vi "Dresden R2R Sputter 03.02.2018 IY24.vi"() -> ()   [LabVIEW 2009] (continued)
                                n25886 = Or(x=w31134, y=w31133) -> (x .or. y?=w31132:bool)
                                }
                                }
                                frame #1 {
                                }
                                }
                                }
                                frame #8 {
                                n25887 = local read "Semi"() -> (w31142:bool)
                                n25888 = case shown="False" w31142 {
                                frame #0 {
                                n25889 = while {
                                i -> [w31143]
                                stop <- w31147 stop-if-true
                                n25890 = Greater?(x=w31143, y=50) -> (0:w31145:bool)
                                n25891 = case shown="True" w31145 {
                                frame #0 {
                                }
                                frame #1 {
                                n25892 = local write "Error Message"("Transfer process was\ncancelled.Please check left limit sensor." ("Error Message")) -> ()
                                n25893 = local write "Semi"(TRUE ("Semi")) -> ()
                                }
                                }
                                n25894 = local read "Cnt_Left_limit_di"() -> (w31149:bool)
                                n25895 = case shown="False" w31149 {
                                tunnel: [FALSE ("Ch1_pet_cool_up_do") TRUE ("Ch1_pet_cool_up_do")] -> w31148
                                frame #0 {
                                n25896 = local write "Cnt_Left_limit_do"(TRUE ("Ch1_pet_cool_up_do")) -> ()
                                n25897 = Wait Until Next ms Multiple(millisecond multiple=u32 200) -> ()  [unwired: 1 out]
                                }
                                frame #1 {
                                }
                                }
                                n25898 = local read "Semi"() -> (w31146:bool)
                                n25899 = Or(x=w31148, y=w31146) -> (x .or. y?=w31147:bool)
                                }
                                }
                                frame #1 {
                                }
                                }
                                }
                                }
                                }
                                frame #1 {
                                }
                                }
                                }
                                frame #1 {
                                n25900 = local read "Semi"() -> (w31156:bool)
                                n25901 = case shown="False" w31156 {
                                frame #0 {
                                n25902 = while {
                                i -> [w31162]
                                stop <- w31159 stop-if-true
                                n25903 = Greater?(x=w31162, y=50) -> (0:w31161:bool)
                                n25904 = case shown="True" w31161 {
                                frame #0 {
                                }
                                frame #1 {
                                n25905 = local write "Error Message"("" ("Error Message")) -> ()
                                n25906 = local write "Semi"(TRUE ("Semi")) -> ()
                                }
                                }
                                n25907 = local read "Casette_servo_start/stop_di"() -> (w31158:bool)
                                n25908 = case shown="False" w31158 {
                                tunnel: [FALSE TRUE] -> w31157
                                frame #0 {
                                n25909 = local write "Casette_servo_start/stop_do"(TRUE ("Casette_servo_left_direction_do")) -> ()
                                n25910 = Wait Until Next ms Multiple(millisecond multiple=u32 500) -> ()  [unwired: 1 out]
                                }
                                frame #1 {
                                }
                                }
                                n25911 = local read "Semi"() -> (w31160:bool)
                                n25912 = Or(x=w31157, y=w31160) -> (x .or. y?=w31159:bool)
                                }
                                }
                                frame #1 {
                                }
                                }
                                }
                                frame #2 {
                                n25913 = local read "Semi"() -> (w31170:bool)
                                n25914 = case shown="False" w31170 {
                                frame #0 {
                                n25915 = while {
                                i -> [w31176]
                                stop <- w31173 stop-if-true
                                n25916 = Greater?(x=w31176, y=50) -> (0:w31175:bool)
                                n25917 = case shown="True" w31175 {
                                frame #0 {
                                }
                                frame #1 {
                                n25918 = local write "Error Message"("" ("Error Message")) -> ()
                                n25919 = local write "Semi"(TRUE ("Semi")) -> ()
                                }
                                }
                                n25920 = local read "Casette_servo_left_direction_di"() -> (w31172:bool)
                                n25921 = case shown="False" w31172 {
                                tunnel: [FALSE TRUE] -> w31171
                                frame #0 {
                                n25922 = local write "Casette_servo_left_direction_do"(TRUE ("Casette_servo_left_direction_do")) -> ()
                                n25923 = Wait Until Next ms Multiple(millisecond multiple=u32 200) -> ()  [unwired: 1 out]
                                }
                                frame #1 {
                                }
                                }
                                n25924 = local read "Semi"() -> (w31174:bool)
                                n25925 = Or(x=w31171, y=w31174) -> (x .or. y?=w31173:bool)
                                }
                                }
                                frame #1 {
                                }
                                }
                                }
                                frame #3 {
                                # "casette motion"
                                n25926 = while {
                                i -> [w31186]
                                stop <- w31184 stop-if-true
                                n25927 = Greater?(x=w31186, y=200) -> (0:w31187:bool)
                                n25928 = case shown="True" w31187 {
                                frame #0 {
                                }
                                frame #1 {
                                n25929 = local write "Semi"(TRUE ("Semi")) -> ()
                                }
                                }
                                n25930 = local read "Counter_read_data"() -> (w31192:i16)
                                n25931 = Greater?(x=w31192, y=i16 0) -> (0:w31190:bool)
                                n25932 = case shown="True" w31190 {
                                tunnel: [TRUE TRUE] -> w31189
                                frame #0 {
                                }
                                frame #1 {
                                n25933 = local write "Casette_servo_start/stop_do"(FALSE ("Casette_servo_start/stop_do")) -> ()
                                n25934 = Wait Until Next ms Multiple(millisecond multiple=u32 200) -> ()  [unwired: 1 out]
                                }
                                }
                                n25935 = local read "Semi"() -> (w31188:bool)
                                n25936 = Or(x=w31189, y=w31188) -> (x .or. y?=w31184:bool)
                                }
                                }
                                frame #4 {
                                n25937 = local read "Semi"() -> (w31198:bool)
                                n25938 = case shown="False" w31198 {
                                frame #0 {
                                n25939 = while {
                                i -> [w31204]
                                stop <- w31201 stop-if-true
                                n25940 = Greater?(x=w31204, y=50) -> (0:w31203:bool)
                                n25941 = case shown="True" w31203 {
                                frame #0 {
                                }
                                frame #1 {
                                n25942 = local write "Error Message"("" ("Error Message")) -> ()
                                n25943 = local write "Semi"(TRUE ("Semi")) -> ()
                                }
                                }
                                n25944 = local read "Casette_servo_start/stop_di"() -> (w31200:bool)
                                n25945 = case shown="True" w31200 {
                                tunnel: [TRUE FALSE] -> w31199
                                frame #0 {
                                }
                                frame #1 {
                                n25946 = local write "Casette_servo_start/stop_do"(FALSE ("Casette_servo_left_direction_do")) -> ()
                                n25947 = Wait Until Next ms Multiple(millisecond multiple=u32 500) -> ()  [unwired: 1 out]
                                }
                                }
                                n25948 = local read "Semi"() -> (w31202:bool)
                                n25949 = Or(x=w31199, y=w31202) -> (x .or. y?=w31201:bool)
                                }
                                }
                                frame #1 {
                                }
                                }
                                }
                                frame #5 {
                                n25950 = local read "Semi"() -> (w31212:bool)
                                n25951 = case shown="False" w31212 {
                                frame #0 {
                                n25952 = Wait (ms)(milliseconds to wait=u32 5000 ("millisecond multiple 2")) -> ()  [unwired: 1 out]
                                }
                                frame #1 {
                                }
                                }
                                }
                                frame #6 {
                                n25953 = local read "Semi"() -> (w31214:bool)
                                n25954 = case shown="False" w31214 {
                                frame #0 {
                                n25955 = while {
                                i -> [w31220]
                                stop <- w31217 stop-if-true
                                n25956 = Greater?(x=w31220, y=50) -> (0:w31219:bool)
                                n25957 = case shown="True" w31219 {
                                frame #0 {
                                }
                                frame #1 {
                                n25958 = local write "Error Message"("" ("Error Message")) -> ()
                                n25959 = local write "Semi"(TRUE ("Semi")) -> ()
                                }
                                }
                                n25960 = local read "Casette_servo_start/stop_di"() -> (w31216:bool)
                                n25961 = case shown="False" w31216 {
                                tunnel: [FALSE TRUE] -> w31215
                                frame #0 {
                                n25962 = local write "Casette_servo_start/stop_do"(TRUE ("Casette_servo_left_direction_do")) -> ()
                                n25963 = Wait Until Next ms Multiple(millisecond multiple=u32 500) -> ()  [unwired: 1 out]
                                }
                                frame #1 {
                                }
                                }
                                n25964 = local read "Semi"() -> (w31218:bool)
                                n25965 = Or(x=w31215, y=w31218) -> (x .or. y?=w31217:bool)
                                }
                                }
                                frame #1 {
                                }
                                }
                                }
                                frame #7 {
                                n25966 = local read "Semi"() -> (w31228:bool)
                                n25967 = case shown="False" w31228 {
                                frame #0 {
                                n25968 = while {
                                i -> [w31234]
                                stop <- w31231 stop-if-true
                                n25969 = Greater?(x=w31234, y=50) -> (0:w31233:bool)
                                n25970 = case shown="True" w31233 {
                                frame #0 {
                                }
                                frame #1 {
                                n25971 = local write "Error Message"("" ("Error Message")) -> ()
                                n25972 = local write "Semi"(TRUE ("Semi")) -> ()
                                }
                                }
                                n25973 = local read "Casette_servo_left_direction_di"() -> (w31230:bool)
                                n25974 = case shown="True" w31230 {
                                tunnel: [TRUE FALSE] -> w31229
                                frame #0 {
                                }
                                frame #1 {
                                n25975 = local write "Casette_servo_left_direction_do"(FALSE ("Casette_servo_left_direction_do")) -> ()
                                n25976 = Wait Until Next ms Multiple(millisecond multiple=u32 200) -> ()  [unwired: 1 out]
                                }
                                }
                                n25977 = local read "Semi"() -> (w31232:bool)
                                n25978 = Or(x=w31229, y=w31232) -> (x .or. y?=w31231:bool)
                                }
                                }
                                frame #1 {
                                }
                                }
                                }
                                frame #8 {
                                # "casette motion"
                                n25979 = while {
                                i -> [w31245]
                                stop <- w31242 stop-if-true
                                n25980 = Greater?(x=w31245, y=200) -> (0:w31246:bool)
                                n25981 = case shown="True" w31246 {
                                frame #0 {
                                }
                                frame #1 {
                                n25982 = local write "Semi"(TRUE ("Semi")) -> ()
                                }
                                }
                                n25983 = local read "Counter_read_data"() -> (w31250:i16)
                                n25984 = Less?(x=w31250, y=i16 0) -> (x < y?=w31249:bool)
                                n25985 = case shown="True" w31249 {
                                tunnel: [TRUE TRUE] -> w31248
                                frame #0 {
                                }
                                frame #1 {
                                n25986 = local write "Casette_servo_start/stop_do"(FALSE ("Casette_servo_start/stop_do")) -> ()
                                n25987 = Wait Until Next ms Multiple(millisecond multiple=u32 200) -> ()  [unwired: 1 out]
                                }
                                }
                                n25988 = local read "Semi"() -> (w31247:bool)
                                n25989 = Or(x=w31248, y=w31247) -> (x .or. y?=w31242:bool)
                                }
                                }
                                frame #9 {
                                n25990 = local read "Semi"() -> (w31256:bool)
                                n25991 = case shown="False" w31256 {
                                frame #0 {
                                n25992 = while {
                                i -> [w31262]
                                stop <- w31259 stop-if-true
                                n25993 = Greater?(x=w31262, y=50) -> (0:w31261:bool)
                                n25994 = case shown="True" w31261 {
                                frame #0 {
                                }
                                frame #1 {
                                n25995 = local write "Error Message"("" ("Error Message")) -> ()
                                n25996 = local write "Semi"(TRUE ("Semi")) -> ()
                                }
                                }
                                n25997 = local read "Casette_servo_start/stop_di"() -> (w31258:bool)
                                n25998 = case shown="True" w31258 {
                                tunnel: [TRUE FALSE] -> w31257
                                frame #0 {
                                }
                                frame #1 {
                                n25999 = local write "Casette_servo_start/stop_do"(FALSE ("Casette_servo_left_direction_do")) -> ()
                                n26000 = Wait Until Next ms Multiple(millisecond multiple=u32 500) -> ()  [unwired: 1 out]
                                }
                                }
                                n26001 = local read "Semi"() -> (w31260:bool)
                                n26002 = Or(x=w31257, y=w31260) -> (x .or. y?=w31259:bool)
                                }
                                }
                                frame #1 {
                                }
                                }
                                }
                                frame #10 {
                                n26003 = local read "Semi"() -> (w31270:bool)
                                n26004 = case shown="False" w31270 {
                                frame #0 {
                                n26005 = local write "SDC1 21b"(TRUE ("SDC1 21b")) -> ()
                                }
                                frame #1 {
                                }
                                }
                                }
                                }
                                }
                                frame #1 {
                                }
                                }
                                }
                                frame #1 {
                                }
                                }
                                }
                                }
                                }
                                frame #1 {
                                }
                                }
                                }
                                frame #1 {
                                n26006 = local read "Semi"() -> (w31272:bool)
                                n26007 = case shown="False" w31272 {
                                frame #0 {
                                n26008 = Wait (ms)(milliseconds to wait=u32 1000) -> ()  [unwired: 1 out]
                                n26009 = local write "SDC1 21"(TRUE ("SDC1 21")) -> ()
                                }
                                frame #1 {
                                }
                                }
                                }
                                }
                                }
                                frame #18 {
                                # "tm parameter"
                                n26010 = local read "Semi"() -> (w31275:bool)
                                n26011 = case shown="False" w31275 {
                                frame #0 {
                                n26012 = local read "Thickness_Monitor_Active"() -> (w31276:bool)
                                n26013 = case shown="True" w31276 {
                                frame #0 {
                                }
                                frame #1 {
                                n26014 = local read "Semi"() -> (w31277:bool)
                                n26015 = case shown="False" w31277 {
                                frame #0 {
                                n26016 = stacked-sequence {
                                frame #0 {
                                n26017 = local read "Semi"() -> (w31278:bool)
                                n26018 = case shown="False" w31278 {
                                frame #0 {
                                n26019 = local read "R Toooling_factor"() -> (w31279:dbl)
                                n26020 = local read "R Material_density"() -> (w31281:dbl)
                                n26021 = local read "R Z_factor"() -> (w31280:dbl)
                                n26022 = local write "Tooling_factor1"(w31279) -> ()
                                n26023 = local write "Material_density"(w31281) -> ()
                                n26024 = local write "Z_factor"(w31280) -> ()
                                }
                                frame #1 {
                                }
                                }
                                }
                                frame #1 {
                                n26025 = local read "Semi"() -> (w31282:bool)
                                n26026 = case shown="False" w31282 {
                                frame #0 {
                                n26027 = Wait (ms)(milliseconds to wait=u32 1000) -> ()  [unwired: 1 out]
                                }
                                frame #1 {
                                }
                                }
                                }
                                frame #2 {
                                n26028 = local read "Semi"() -> (w31284:bool)
                                n26029 = case shown="False" w31284 {
                                frame #0 {
                                n26030 = local read "R Single DC Target material"() -> (w31285:string)
                                n26031 = Write to Text File(file (use dialog)=path path "D/VK-1701 System Files/Material Data/data1.txt", text=w31285) -> ()  [unwired: 2 in, 3 out]
                                }
                                frame #1 {
                                }
                                }
                                }
                                frame #3 {
                                n26032 = local read "Semi"() -> (w31287:bool)
                                n26033 = case shown="False" w31287 {
                                frame #0 {
                                n26034 = local write "SDC1 22"(TRUE ("SDC1 22")) -> ()
                                n26035 = Wait (ms)(milliseconds to wait=u32 1000) -> ()  [unwired: 1 out]
                                }
                                frame #1 {
                                }
                                }
                                }
                                }
                                }
                                frame #1 {
                                }
                                }
                                }
                                }
                                }
                                frame #1 {
                                }
                                }
                                }
                                frame #19 {
                                n26036 = local read "Semi"() -> (w31290:bool)
                                n26037 = case shown="False" w31290 {
                                frame #0 {
                                n26038 = local read "R_Web_selection"() -> (w31291:enum32{"Web", "Other"})
                                n26039 = case shown="\"Other\"" w31291 {
                                frame #0 {
                                }
                                frame #1 {
                                n26040 = local read "R_Thickness Selection"() -> (w31292:enum32{"Thickness", "Time"})
                                n26041 = case shown="\"Thickness\", Default" w31292 {
                                frame #0 {
                                n26042 = local read "Semi"() -> (w31295:bool)
                                n26043 = case shown="False" w31295 {
                                frame #0 {
                                n26044 = stacked-sequence {
                                frame #0 {
                                n26045 = local read "Semi"() -> (w31296:bool)
                                n26046 = case shown="False" w31296 {
                                frame #0 {
                                n26047 = local write "Tm1_auto_set_zero"(TRUE ("Tm1_auto_set_zero")) -> ()
                                n26048 = Wait (ms)(milliseconds to wait=u32 3000) -> ()  [unwired: 1 out]
                                }
                                frame #1 {
                                }
                                }
                                }
                                frame #1 {
                                n26049 = local read "Semi"() -> (w31299:bool)
                                n26050 = case shown="False" w31299 {
                                frame #0 {
                                n26051 = flat-sequence {
                                frame #0 {
                                n26052 = local write "Process_sputter"(u8 0 ("Process_sputter")) -> ()
                                }
                                frame #1 {
                                n26053 = Wait (ms)(milliseconds to wait=u32 1000) -> ()  [unwired: 1 out]
                                }
                                }
                                }
                                frame #1 {
                                }
                                }
                                }
                                frame #2 {
                                n26054 = local read "Semi"() -> (w31302:bool)
                                n26055 = case shown="False" w31302 {
                                frame #0 {
                                n26056 = property on="Process_tab_sputter" class="TabCtl (strict)"("Visible"=TRUE) -> ()  [unwired: 2 in, 2 out]
                                n26057 = local write "Process_sputter"(u8 0 ("Process_sputter")) -> ()
                                }
                                frame #1 {
                                }
                                }
                                }
                                frame #3 {
                                n26058 = local read "Semi"() -> (w31305:bool)
                                n26059 = case shown="False" w31305 {
                                frame #0 {
                                n26060 = while {
                                stop <- w31310 stop-if-true
                                n26061 = local read "R_Target Thickness Value"() -> (w31308:dbl)
                                n26062 = local read "Thickness 1-1"() -> (w31307:dbl)
                                n26063 = local read "Tm1_fail"() -> (w31318:bool)
                                n26064 = case shown="True" w31318 {
                                tunnel: [FALSE TRUE] -> w31311
                                frame #0 {
                                }
                                frame #1 {
                                n26065 = local write "Error Message"("Sputtering Process cancelled.\nPlease check TM1 connections." ("Error Message")) -> ()
                                }
                                }
                                n26066 = Divide(x=w31307, y=w31308) -> (x/y=w31316:dbl)
                                n26067 = Multiply(x=w31316, y=100.0) -> (x*y=w31314:dbl)
                                n26068 = Greater Or Equal?(x=w31314, y=100.0) -> (x >= y?=w31313:bool)
                                n26069 = local write "Target Thickness Sputter"(w31308) -> ()
                                n26070 = local write "Thickness_total"(w31307) -> ()
                                n26071 = local read "Abort_sputter"() -> (w31306:bool)
                                n26072 = local write "Process_sputter"(w31314) -> ()
                                n26073 = Wait Until Next ms Multiple(millisecond multiple=u32 300) -> ()  [unwired: 1 out]
                                n26074 = local read "Semi"() -> (w31312:bool)
                                n26075 = Compound Arithmetic op=OR(w31312, w31313, w31306, w31311) -> (w31310:bool)
                                }
                                }
                                frame #1 {
                                }
                                }
                                }
                                frame #4 {
                                n26076 = local read "Semi"() -> (w31322:bool)
                                n26077 = case shown="False" w31322 {
                                frame #0 {
                                w31323 = FALSE ("Abort_sputter")
                                n26078 = property on="Process_tab_sputter" class="TabCtl (strict)"("Visible"=w31323) -> ()  [unwired: 2 in, 2 out]
                                n26079 = local write "Abort_sputter"(w31323) -> ()
                                }
                                frame #1 {
                                }
                                }
                                }
                                frame #5 {
                                n26080 = local read "Tm1_fail"() -> (w31324:bool)
                                n26081 = case shown="False" w31324 {
                                frame #0 {
                                n26082 = Wait (ms)(milliseconds to wait=u32 1000) -> ()  [unwired: 1 out]
                                n26083 = local write "SDC1 23"(TRUE ("SDC1 23")) -> ()
                                }
                                frame #1 {
                                }
                                }
                                }
                                }
                                }
                                frame #1 {
                                }
                                }
                                }
                                frame #1 {
                                n26084 = local read "Semi"() -> (w31327:bool)
                                n26085 = case shown="False" w31327 {
                                frame #0 {
                                n26086 = stacked-sequence {
                                frame #0 {
                                n26087 = local read "Semi"() -> (w31328:bool)
                                n26088 = case shown="False" w31328 {
                                frame #0 {
                                w31329 = TRUE ("Tm1_auto_set_zero")
                                n26089 = local write "Tm1_auto_set_zero"(w31329) -> ()
                                n26090 = property on="Sputter_tab" class="TabCtl (strict)"("Visible"=w31329) -> ()  [unwired: 2 in, 2 out]
                                n26091 = Wait (ms)(milliseconds to wait=u32 1000) -> ()  [unwired: 1 out]
                                }
                                frame #1 {
                                }
                                }
                                }
                                frame #1 {
                                n26092 = local read "Semi"() -> (w31331:bool)
                                n26093 = case shown="False" w31331 {
                                frame #0 {
                                n26094 = while {
                                i -> [w31340]
                                stop <- w31339 stop-if-true
                                n26095 = Wait Until Next ms Multiple(millisecond multiple=u32 1000) -> ()  [unwired: 1 out]
                                n26096 = local read "R_Duration"() -> (w31341:dbl)
                                n26097 = local read "Sputter_cancel"() -> (w31332:bool)
                                n26098 = local read "Semi"() -> (w31336:bool)
                                n26099 = Multiply(x=w31341, y=60.0) -> (x*y=w31338:dbl)
                                n26100 = Greater?(x=w31340, y=w31338) -> (0:w31337:bool)
                                n26101 = Compound Arithmetic op=OR(w31336, w31332, w31337) -> (w31335:bool)
                                n26102 = local read "R_Duration"() -> (w31333:dbl)
                                n26103 = case shown="False" w31335 {
                                tunnel: w31340 -> [w31345 _]
                                tunnel: [FALSE TRUE] -> w31339
                                tunnel: w31338 -> [w31346 _]
                                frame #0 {
                                n26104 = Subtract(x=w31346, y=w31345) -> (x-y=w31343:dbl)
                                n26105 = local write "Sputter_left_time"(w31343) -> ()
                                }
                                frame #1 {
                                n26106 = property on="Sputter_tab" class="TabCtl (strict)"("Visible"=FALSE) -> ()  [unwired: 2 in, 2 out]
                                }
                                }
                                n26107 = local write "Sputter_set_time"(w31333) -> ()
                                }
                                }
                                frame #1 {
                                }
                                }
                                }
                                frame #2 {
                                n26108 = local write "Sputter_cancel"(FALSE ("Sputter_cancel")) -> ()
                                }
                                frame #3 {
                                n26109 = local write "SDC1 24"(TRUE ("SDC1 24")) -> ()
                                n26110 = Wait (ms)(milliseconds to wait=u32 1000) -> ()  [unwired: 1 out]
                                }
                                }
                                }
                                frame #1 {
                                }
                                }
                                }
                                }
                                n26111 = local read "Substrate Material"() -> (w31293:string)
                                n26112 = Write to Text File(file (use dialog)=path path "D/VK-1701 System Files/Material Data/data2.txt", text=w31293) -> ()  [unwired: 2 in, 3 out]
                                }
                                }
                                }
                                frame #1 {
                                }
                                }
                                }
                                frame #20 {
                                # "CLOSE DC"
                                n26113 = local read "Semi"() -> (w31352:bool)
                                n26114 = case shown="False" w31352 {
                                frame #0 {
                                n26115 = stacked-sequence {
                                frame #0 {
                                n26116 = local read "Semi"() -> (w31353:bool)
                                n26117 = case shown="False" w31353 {
                                frame #0 {
                                n26118 = local write "Dc_auto_off"(TRUE ("Dc_auto_off")) -> ()
                                }
                                frame #1 {
                                }
                                }
                                }
                                frame #1 {
                                n26119 = local read "Semi"() -> (w31355:bool)
                                n26120 = case shown="False" w31355 {
                                frame #0 {
                                n26121 = Wait (ms)(milliseconds to wait=u32 1000) -> ()  [unwired: 1 out]
                                }
                                frame #1 {
                                }
                                }
                                }
                                frame #2 {
                                n26122 = local read "Semi"() -> (w31357:bool)
                                n26123 = case shown="False" w31357 {
                                frame #0 {
                                n26124 = local write "Dc_auto_set_zero"(TRUE ("Dc_auto_set")) -> ()
                                }
                                frame #1 {
                                }
                                }
                                }
                                frame #3 {
                                n26125 = local read "Semi"() -> (w31359:bool)
                                n26126 = case shown="False" w31359 {
                                frame #0 {
                                n26127 = Wait (ms)(milliseconds to wait=u32 1000) -> ()  [unwired: 1 out]
                                }
                                frame #1 {
                                }
                                }
                                }
                                frame #4 {
                                n26128 = local read "Semi"() -> (w31361:bool)
                                n26129 = case shown="False" w31361 {
                                frame #0 {
                                n26130 = while {
                                i -> [w31373]
                                stop <- w31362 stop-if-true
                                n26131 = Greater?(x=w31373, y=600) -> (0:w31372:bool)
                                n26132 = case shown="True" w31372 {
                                frame #0 {
                                }
                                frame #1 {
                                n26133 = local write "Semi"(TRUE ("Semi")) -> ()
                                n26134 = local write "Error Message"("Sputter Process cancelled.\nPlease Check DC connections." ("Error Message")) -> ()
                                }
                                }
                                n26135 = local read "Actual DC Power"() -> (w31367:dbl)
                                n26136 = local read "Actual DC Volt :"() -> (w31366:dbl)
                                n26137 = Less?(x=w31367, y=10.0) -> (x < y?=w31370:bool)
                                n26138 = Less?(x=w31366, y=20.0) -> (x < y?=w31371:bool)
                                n26139 = And(x=w31370, y=w31371) -> (x .and. y?=w31364:bool)
                                n26140 = local read "Semi"() -> (w31363:bool)
                                n26141 = Wait Until Next ms Multiple(millisecond multiple=u32 500) -> ()  [unwired: 1 out]
                                n26142 = Compound Arithmetic op=OR(w31364, w31363) -> (w31362:bool)
                                }
                                }
                                frame #1 {
                                }
                                }
                                }
                                frame #5 {
                                n26143 = local read "Semi"() -> (w31377:bool)
                                n26144 = case shown="False" w31377 {
                                frame #0 {
                                n26145 = while {
                                i -> [w31383]
                                stop <- w31378 stop-if-true
                                n26146 = Greater?(x=w31383, y=50) -> (0:w31382:bool)
                                n26147 = case shown="True" w31382 {
                                frame #0 {
                                }
                                frame #1 {
                                n26148 = local write "Semi"(TRUE ("Semi")) -> ()
                                n26149 = local write "Error Message"("Sputter Process cancelled.\nPlease Check DCPS-SW1." ("Error Message")) -> ()
                                }
                                }
                                n26150 = local read "Cnt_Dcps_sw1_di"() -> (w31381:bool)
                                n26151 = case shown="False" w31381 {
                                tunnel: [TRUE ("Cnt_Dcps_sw1_do") FALSE ("Cnt_Dcps_sw1_do")] -> w31380
                                frame #0 {
                                }
                                frame #1 {
                                n26152 = local write "Cnt_Dcps_sw1_do"(FALSE ("Cnt_Dcps_sw1_do")) -> ()
                                n26153 = Wait Until Next ms Multiple(millisecond multiple=u32 500) -> ()  [unwired: 1 out]
                                }
                                }
                                n26154 = local read "Semi"() -> (w31379:bool)
                                n26155 = Or(x=w31380, y=w31379) -> (x .or. y?=w31378:bool)
                                }
                                }
                                frame #1 {
                                }
                                }
                                }
                                frame #6 {
                                n26156 = local read "Semi"() -> (w31391:bool)
                                n26157 = case shown="False" w31391 {
                                frame #0 {
                                n26158 = Wait (ms)(milliseconds to wait=u32 1000) -> ()  [unwired: 1 out]
                                n26159 = local write "SDC1 25"(TRUE ("SDC1 25")) -> ()
                                }
                                frame #1 {
                                }
                                }
                                }
                                }
                                }
                                frame #1 {
                                }
                                }
                                }
                                frame #21 {
                                # "PC-BV OPEN"
                                n26160 = stacked-sequence {
                                frame #0 {
                                n26161 = local read "Semi"() -> (w31394:bool)
                                n26162 = case shown="False" w31394 {
                                frame #0 {
                                n26163 = stacked-sequence {
                                frame #0 {
                                n26164 = local read "Semi"() -> (w31395:bool)
                                n26165 = case shown="False" w31395 {
                                frame #0 {
                                n26166 = local write "Pc_bv2_auto_open"(TRUE ("Tp1_auto_start")) -> ()
                                }
                                frame #1 {
                                }
                                }
                                }
                                frame #1 {
                                n26167 = local read "Semi"() -> (w31397:bool)
                                n26168 = case shown="False" w31397 {
                                frame #0 {
                                n26169 = Wait (ms)(milliseconds to wait=u32 1000) -> ()  [unwired: 1 out]
                                }
                                frame #1 {
                                }
                                }
                                }
                                frame #2 {
                                n26170 = local read "Semi"() -> (w31399:bool)
                                n26171 = case shown="False" w31399 {
                                frame #0 {
                                n26172 = while {
                                i -> [w31405]
                                stop <- w31401 stop-if-true
                                n26173 = local read "Pc_bv_opened_ch2"() -> (w31403:bool)
                                n26174 = Greater?(x=w31405, y=120) -> (0:w31404:bool)
                                n26175 = local read "Semi"() -> (w31402:bool)
                                n26176 = Compound Arithmetic op=OR(w31402, w31403, w31404) -> (w31401:bool)
                                n26177 = Wait (ms)(milliseconds to wait=u32 500) -> ()  [unwired: 1 out]
                                }
                                }
                                frame #1 {
                                }